vi "CRYO_MASTER_FULL_RUN3.vi"() -> ()   [LabVIEW 2017]
uses:
  LSI218Data.lvclass
  LSI336Data.lvclass
  USBData.lvclass
  6240AData.lvclass
  DMMsData.lvclass
  LMData.lvclass
  <vilib>/DAQmx/miscellaneous.llb/DAQmx Fill In Error Info.vi
  <vilib>/DAQmx/create/channels.llb/DAQmx Create Channel (DO-Digital Output).vi
  <vilib>/DAQmx/create/channels.llb/DAQmx Create Channel (AO-Voltage-Basic).vi
  <vilib>/express/express arith-compare/Formula/XNode/ExpressFormulaBlockNode.xnode
  <vilib>/Analysis/NI_AALBase.lvlib
  istr.lib/Agilent 33XXX Series/Agilent 33XXX Series.lvlib
panel:
  in  "Automatic \nScreenshots?":bool=TRUE
  in  "Frontpanel screenshots":bool
  in  "Screenshots interval":i64=3605
  in  "Record interval":i64=20
  out "Cycle #":u32=1
  in  "Measurement Interval (s)":dbl=1.0
  in  "Stop Button":bool
  in  "?":T1(tab)=enum."MEASUREMENT"
  out "RUN Identifier":string="20210209_084357_RUNIII"
  in  "Base Path (screenshots)":path=path "C:/LabVIEW/DATA/Google/TUCAN Experiments/KEK_cryotests_2019-2020/data/screenshots"
  out "error out (USB6210/6218 AOUT)":errorcluster
  in  "AOUT Labels":string[](array[string])=["PWR400H_I", "PMC183A_I"]
  in  "DOUT Labels":string[](array[string])=["D_V1_NO", "D_V2_NC", "D_CV1", "D_H1"]
  in  "AOUT assignment":tag[](array[tag])=["Dev1/ao0", "Dev1/ao1"]
  out "AO task out":refnum<k21>="20210209_084357_RUNIII_AO"
  in  "Analog Out ON?":bool=TRUE
  in  "InstName (USB6218)":string="USB6218"
  in  "USB6218 Config":T2(array[cluster])=[{"Label"="F_1", "FileFormat"="%5.5f", "Active?"=TRUE, "Physical CH"="Dev1/ai0", " terminal\n type"=10083, "ConversionType"={"Type"=enum."SimpleProp", "ConversionParameters"=[0.0, 5.0, 0.0, 500.0]}, "VoltageLimits"=[0.0, 5.0]}, {"Label"="F_2", "FileFormat"="%5.5f", "Active?"=TRUE, "Physical CH"="Dev1/ai1", " terminal\n type"=10083, "ConversionType"={"Type"=enum."SimpleProp", "ConversionParameters"=[0.0, 5.0, 0.0, 200.0]}, "VoltageLimits"=[0.0, 5.0]}, {"Label"="F_3", "FileFormat"="%5.5f", "Active?"=TRUE, "Physical CH"="Dev1/ai2", " terminal\n type"=10083, "ConversionType"={"Type"=enum."SimpleProp", "ConversionParameters"=[0.0, 5.0, 0.0, 200.0]}, "VoltageLimits"=[0.0, 5.0]}, {"Label"="F_4", "FileFormat"="%5.5f", "Active?"=TRUE, "Physical CH"="Dev1/ai3", " terminal\n type"=10083, "ConversionType"={"Type"=enum."SimpleProp", "ConversionParameters"=[0.0, 5.0, 0.0, 500.0]}, "VoltageLimits"=[0.0, 5.0]}, {"Label"="F_5", "FileFormat"="%5.5f", "Active?"=TRUE, "Physical CH"="Dev1/ai4", " terminal\n type"=10083, "ConversionType"={"Type"=enum."SimpleProp", "ConversionParameters"=[0.0, 5.0, 0.0, 500.0]}, "VoltageLimits"=[0.0, 5.0]}, {"Label"="I_CV", "FileFormat"="%3.5f", "Active?"=TRUE, "Physical CH"="Dev1/ai5", " terminal\n type"=10083, "ConversionType"={"Type"=enum."Raw", "ConversionParameters"=[0.0, 0.0, 0.0, 0.0]}, "VoltageLimits"=[0.0, 10.0]}, {"Label"="CV1_answer", "FileFormat"="%3.5f", "Active?"=TRUE, "Physical CH"="Dev1/ai6", " terminal\n type"=10083, "ConversionType"={"Type"=enum."SimpleProp", "ConversionParameters"=[1.0, 5.0, 0.0, 100.0]}, "VoltageLimits"=[0.0, 5.0]}, {"Label"="P_Dewar", "FileFormat"="%5.5e", "Active?"=TRUE, "Physical CH"="Dev1/ai7", " terminal\n type"=10083, "ConversionType"={"Type"=enum."SimpleProp", "ConversionParameters"=[1.0, 5.0, 0.0, 200000.0]}, "VoltageLimits"=[0.0, 5.0]}, {"Label"="L_Dewar", "FileFormat"="%5.5f", "Active?"=TRUE, "Physical CH"="Dev1/ai8", " terminal\n type"=10083, "ConversionType"={"Type"=enum."SimpleProp", "ConversionParameters"=[0.0, 10.0, 0.0, 100.0]}, "VoltageLimits"=[0.0, 10.0]}] {"terminal\n type" items=["Default"=-1, "RSE"=10083, "NRSE"=10078, "Differential"=10106, "Pseudodifferential"=12529]}
  out "error out (USB6218)":errorcluster
  out "error out (USB6210/6218 DOUT)":errorcluster
  out "DOUT task out":refnum<k21>="20210209_084357_DO"
  in  "DOUT Physical CH":tag[](array[tag])=["Dev1/port1/line0", "Dev1/port1/line1", "Dev1/port1/line2", "Dev1/port1/line3"]
  in  "Digital Out ON?":bool=TRUE
  in  "USB6210 Config":T2(array[cluster])=[{"Label"="P_ins", "FileFormat"="%5.5e", "Active?"=TRUE, "Physical CH"="Dev2/ai0", " terminal\n type"=10083, "ConversionType"={"Type"=enum."CC-10_LOG", "ConversionParameters"=[0.5, 9.0, 0.0, 1.0]}, "VoltageLimits"=[0.0, 10.0]}, {"Label"="P_4Kres", "FileFormat"="%5.5e", "Active?"=TRUE, "Physical CH"="Dev2/ai1", " terminal\n type"=10083, "ConversionType"={"Type"=enum."SimpleProp", "ConversionParameters"=[1.0, 5.0, 0.0, 200000.0]}, "VoltageLimits"=[0.0, 5.0]}, {"Label"="P_3HeIN", "FileFormat"="%5.5e", "Active?"=TRUE, "Physical CH"="Dev2/ai2", " terminal\n type"=10083, "ConversionType"={"Type"=enum."SimpleProp", "ConversionParameters"=[1.0, 5.0, 0.0, 200000.0]}, "VoltageLimits"=[0.0, 5.0]}, {"Label"="P_SldRTN", "FileFormat"="%5.5e", "Active?"=TRUE, "Physical CH"="Dev2/ai3", " terminal\n type"=10083, "ConversionType"={"Type"=enum."SimpleProp", "ConversionParameters"=[1.0, 5.0, 0.0, 200000.0]}, "VoltageLimits"=[0.0, 5.0]}, {"Label"="P_3Hepot", "FileFormat"="%5.5e", "Active?"=TRUE, "Physical CH"="Dev2/ai4", " terminal\n type"=10083, "ConversionType"={"Type"=enum."SimpleProp", "ConversionParameters"=[0.0, 10.0, 0.0, 133320.0]}, "VoltageLimits"=[0.0, 10.0]}, {"Label"="P_1Kpot", "FileFormat"="%5.5e", "Active?"=TRUE, "Physical CH"="Dev2/ai5", " terminal\n type"=10083, "ConversionType"={"Type"=enum."SimpleProp", "ConversionParameters"=[0.0, 10.0, 0.0, 133320.0]}, "VoltageLimits"=[0.0, 10.0]}, {"Label"="P_Dewar(old)", "FileFormat"="%5.5e", "Active?"=FALSE, "Physical CH"="Dev2/ai6", " terminal\n type"=10083, "ConversionType"={"Type"=enum."SimpleProp", "ConversionParameters"=[1.0, 5.0, 0.0, 200000.0]}, "VoltageLimits"=[0.0, 5.0]}, {"Label"="DP_HEX4", "FileFormat"="%5.5e", "Active?"=TRUE, "Physical CH"="Dev2/ai7", " terminal\n type"=10083, "ConversionType"={"Type"=enum."SimpleProp", "ConversionParameters"=[1.0, 5.0, 0.0, 1000.0]}, "VoltageLimits"=[0.0, 5.0]}, {"Label"="DP_HEX5", "FileFormat"="%5.5e", "Active?"=TRUE, "Physical CH"="Dev2/ai8", " terminal\n type"=10083, "ConversionType"={"Type"=enum."SimpleProp", "ConversionParameters"=[1.0, 5.0, 0.0, 1000.0]}, "VoltageLimits"=[0.0, 5.0]}, {"Label"="L1(old)", "FileFormat"="%5.5f", "Active?"=TRUE, "Physical CH"="Dev2/ai9", " terminal\n type"=10083, "ConversionType"={"Type"=enum."SimpleProp", "ConversionParameters"=[0.0, 10.0, 0.0, 100.0]}, "VoltageLimits"=[0.0, 10.0]}, {"Label"="L2-1", "FileFormat"="%5.5f", "Active?"=TRUE, "Physical CH"="Dev2/ai10", " terminal\n type"=10083, "ConversionType"={"Type"=enum."SimpleProp", "ConversionParameters"=[0.0, 10.0, 0.0, 100.0]}, "VoltageLimits"=[0.0, 10.0]}, {"Label"="L2-2", "FileFormat"="%5.5f", "Active?"=TRUE, "Physical CH"="Dev2/ai11", " terminal\n type"=10083, "ConversionType"={"Type"=enum."SimpleProp", "ConversionParameters"=[0.0, 10.0, 0.0, 100.0]}, "VoltageLimits"=[0.0, 10.0]}, {"Label"="L3", "FileFormat"="%5.5f", "Active?"=TRUE, "Physical CH"="Dev2/ai12", " terminal\n type"=10083, "ConversionType"={"Type"=enum."SimpleProp", "ConversionParameters"=[0.0, 10.0, 0.0, 100.0]}, "VoltageLimits"=[0.0, 10.0]}, {"Label"="P_HEX7OUT", "FileFormat"="%5.5e", "Active?"=TRUE, "Physical CH"="Dev2/ai13", " terminal\n type"=10083, "ConversionType"={"Type"=enum."SimpleProp", "ConversionParameters"=[1.0, 5.0, 0.0, 200000.0]}, "VoltageLimits"=[0.0, 5.0]}, {"Label"="P_IP", "FileFormat"="%5.5e", "Active?"=TRUE, "Physical CH"="Dev2/ai14", " terminal\n type"=10083, "ConversionType"={"Type"=enum."CC-10_LOG", "ConversionParameters"=[0.5, 9.0, 0.0, 1.0]}, "VoltageLimits"=[0.0, 10.0]}, {"Label"="V_H1", "FileFormat"="%3.5f", "Active?"=TRUE, "Physical CH"="Dev2/ai15", " terminal\n type"=10083, "ConversionType"={"Type"=enum."Raw", "ConversionParameters"=[0.0, 1.0, 0.0, 1.0]}, "VoltageLimits"=[0.0, 10.0]}] {"terminal\n type" items=["Default"=-1, "RSE"=10083, "NRSE"=10078, "Differential"=10106, "Pseudodifferential"=12529]}
  in  "RUN label":string="RUNIII"
  in  "Base Path":path=path "C:/LabVIEW/DATA/RUN_3"
  in  "InstName (USB6210)":string="USB6210"
  out "error out (USB6210)":errorcluster
  out "File Refn USB AO":refnum<file>
  out "File Refn USB DO":refnum<file>
  in  "LM measurement interval (>0)":i64=1
  in  "Active? (HP34401 LM)":bool=TRUE
  in  "Labels (HP34401 LM)":string[](array[string])=["R_L1", "L1"]
  in  "FileFormat (HP34401 LM)":string[](array[string])=["%.4f", "%.4f"]
  in  "VISA (HP34401 LM)":refnum<visa-resource-name>="GPIB0::24::INSTR"
  in  "LevelCalibration (R0, R1, L0, L1)":dbl[](array[numeric])=[179.74, 0.0, 0.0, 100.0]
  in  "InstName (HP34401 LM)":string="HP34401LM"
  out "error out (LSI336)":errorcluster
  in  "InstName (LSI336)":string="LSI336"
  in  "FileFormat (336)":string="%4.4f"
  in  "LSI336Settings(X,Y)":T3(array[cluster])=[{"LSIName"="LSi336X", "Labels"=["T1K3-1", "T1K3-2", "T3He5", "T3He8"], "SensorLocations"=[enum."T1K3-1", enum."T1K3-2", enum."T3He5", enum."T3He8"], "Active?"=TRUE, "VISA res. name"="COM15_LSI336Y"}, {"LSIName"="LSi336Y", "Labels"=["T3He6-1", "T3He6-2", "T3He7-1", "T3He7-2"], "SensorLocations"=[enum."T3He6-1", enum."T3He6-2", enum."T3He7-1", enum."T3He7-2"], "Active?"=TRUE, "VISA res. name"="COM20_LSI336X"}]
  in  "FileFormat (218)":string="%4.4f"
  in  "InstName (LSI218)":string="LSI218"
  in  "LSI218Settings(A-F)":T3(array[cluster])=[{"LSIName"="LSI218A", "Labels"=["T3He10", "T3He1-1", "TTH3", "TTH4", "TTH1", "TTH2", "T4He1", "T1K1"], "SensorLocations"=[enum."T3He10", enum."T3He1-1", enum."TTH3", enum."TTH4", enum."TTH1", enum."TTH2", enum."T4He1", enum."T1K1"], "Active?"=TRUE, "VISA res. name"="GPIB0::7::INSTR"}, {"LSIName"="LSI218B", "Labels"=["N.C.", "N.C.", "N.C.", "N.C.", "T3He2-1", "T3He2-2", "T3He3", "T3He1-4"], "SensorLocations"=[enum."N.C.", enum."N.C.", enum."N.C.", enum."N.C.", enum."T3He2-1", enum."T3He2-2", enum."T3He3", enum."T3He1-4"], "Active?"=TRUE, "VISA res. name"="GPIB0::4::INSTR"}, {"LSIName"="LSI218C", "Labels"=["T4He3-1", "T4He3-2", "T4He3-3", "T4He3-4", "T4He2-1", "T4He2-2", "T4He4", "T4He5"], "SensorLocations"=[enum."T4He3-1", enum."T4He3-2", enum."T4He3-3", enum."T4He3-4", enum."T4He2-1", enum."T4He2-2", enum."T4He4", enum."T4He5"], "Active?"=TRUE, "VISA res. name"="GPIB0::3::INSTR"}, {"LSIName"="LSI218D", "Labels"=["T4He6", "T4He9", "T3He1-2", "T3He1-3", "T4He7", "T4He8", "T4He10", "T1K6"], "SensorLocations"=[enum."T4He6", enum."T4He9", enum."T3He1-2", enum."T3He1-3", enum."T4He7", enum."T4He8", enum."T4He10", enum."T1K6"], "Active?"=TRUE, "VISA res. name"="GPIB0::5::INSTR"}, {"LSIName"="LSI218E", "Labels"=["TIP1", "N.C.", "TIP2", "N.C.", "TIP3", "TIP4", "TIP5", "N.C."], "SensorLocations"=[enum."TIP1", enum."N.C.", enum."TIP2", enum."N.C.", enum."TIP3", enum."TIP4", enum."TIP5", enum."N.C."], "Active?"=TRUE, "VISA res. name"="GPIB0::11::INSTR"}, {"LSIName"="LSI218F", "Labels"=["T1K2", "T1K4", "T1K5", "T3He4", "T3He9", "TIP6", "N.C.", "N.C."], "SensorLocations"=[enum."T1K2", enum."T1K4", enum."T1K5", enum."T3He4", enum."T3He9", enum."TIP6", enum."N.C.", enum."N.C."], "Active?"=TRUE, "VISA res. name"="GPIB0::8::INSTR"}]
  out "error out (LSI218)":errorcluster={"status"=TRUE, "code"=-1073807338, "source"="VISA Close in Lake Shore Cryotronics 218.lvlib:Close.vi->LSI218Data.lvclass:LSI218Data_terminate.vi->CRYO_MASTER_FULL_RUN3.vi"}
  out "RUN Identifier 2":string="20210209_084357_RUNIII" caption="RUN Identifier"
  out "error out (HP34401 LM)":errorcluster
  out "Graph 3":T4(graph)=[{"TimeArray"=[timestamp(3695672639.4136896 s since 1904-01-01)], "DataArray"=[-0.36185606613019977]}, {"TimeArray"=[timestamp(3695672639.4136896 s since 1904-01-01)], "DataArray"=[-1.4204433335631088]}, {"TimeArray"=[timestamp(3695672639.4136896 s since 1904-01-01)], "DataArray"=[0.28794373208354185]}, {"TimeArray"=[timestamp(3695672639.4136896 s since 1904-01-01)], "DataArray"=[-3.0973798990583647]}, {"TimeArray"=[timestamp(3695672639.4136896 s since 1904-01-01)], "DataArray"=[18.382396544680894]}, {"TimeArray"=[timestamp(3695672639.4136896 s since 1904-01-01)], "DataArray"=[-0.0024966396874153696]}, {"TimeArray"=[timestamp(3695672639.4136896 s since 1904-01-01)], "DataArray"=[107.20664477077275]}] caption="XY Graph"
  out "Graph 1":T4(graph)=[{"TimeArray"=[timestamp(3695672639.4087214 s since 1904-01-01)], "DataArray"=[18.674861858538797]}, {"TimeArray"=[timestamp(3695672639.4087214 s since 1904-01-01)], "DataArray"=[97865.81349287118]}, {"TimeArray"=[timestamp(3695672639.4087214 s since 1904-01-01)], "DataArray"=[100998.44453584745]}, {"TimeArray"=[timestamp(3695672639.4087214 s since 1904-01-01)], "DataArray"=[100709.02551899779]}, {"TimeArray"=[timestamp(3695672639.4087214 s since 1904-01-01)], "DataArray"=[101407.09548804205]}, {"TimeArray"=[timestamp(3695672639.4087214 s since 1904-01-01)], "DataArray"=[101279.08758660906]}, {"TimeArray"=[timestamp(3695672639.4087214 s since 1904-01-01)], "DataArray"=[0.0]}, {"TimeArray"=[timestamp(3695672639.4087214 s since 1904-01-01)], "DataArray"=[100273.25274306418]}, {"TimeArray"=[timestamp(3695672639.4087214 s since 1904-01-01)], "DataArray"=[4.684755546764993e-05]}, {"TimeArray"=[timestamp(3695672639.4136896 s since 1904-01-01)], "DataArray"=[102243.79868545999]}] caption="XY Graph"
  in  "FIle suffix 4":string="Graph4_noise"
  in  "Take Screenshot! 4":bool
  in  "Take Screenshot! 3":bool
  in  "Take Screenshot! 2":bool
  in  "Take Screenshot! 1":bool
  in  "FIle suffix 3":string="Graph3_noise"
  in  "FIle suffix 2":string="Graph2_noise"
  in  "FIle suffix 1":string="Graph1_noise"
  in  "log/linear 2":bool
  in  "Tab Control 2":T5(tab)
  in  "Plot selecter (USB6210)\n    1      2     3     4":bool[][](array[boolean])=[[TRUE, FALSE, FALSE, FALSE], [TRUE, FALSE, FALSE, FALSE], [TRUE, FALSE, FALSE, FALSE], [TRUE, FALSE, FALSE, FALSE], [TRUE, FALSE, FALSE, FALSE], [TRUE, FALSE, FALSE, FALSE], [TRUE, FALSE, FALSE, FALSE], [FALSE, TRUE, FALSE, FALSE], [FALSE, TRUE, FALSE, FALSE], [FALSE, TRUE, FALSE, FALSE], [FALSE, TRUE, FALSE, FALSE], [FALSE, TRUE, FALSE, FALSE], [FALSE, TRUE, FALSE, FALSE], [TRUE, FALSE, FALSE, FALSE], [TRUE, FALSE, FALSE, FALSE], [FALSE, FALSE, FALSE, FALSE]]
  out "All Labels (USB6210)":string[](array[string])=["P_ins", "P_4Kres", "P_3HeIN", "P_SldRTN", "P_3Hepot", "P_1Kpot", "P_Dewar(old)", "DP_HEX4", "DP_HEX5", "L1(old)", "L2-1", "L2-2", "L3", "P_HEX7OUT", "P_IP", "V_H1"]
  out "Last Data \n(USB6210)":dbl[](array[numeric])=[18.674861858538797, 97865.81349287118, 100998.44453584745, 100709.02551899779, 101407.09548804205, 101279.08758660906, 0.0, -48.20456535494683, 0.06691412080322978, 10.108489682314854, 0.1698011167381339, -0.07483544992953703, 0.04024895650740204, 100273.25274306418, 4.684755546764993e-05, 5.953981760223165] format="%#_6e"
  out "Time of Last Measurement (USB6210)":timestamp=timestamp(3695672639.4087214 s since 1904-01-01)
  out "USB6210 Status":T6(ring)=enum."Ready"
  out "Last Vol\n(USB6210)":dbl[](array[numeric])=[8.135628698970727, 2.9573162698574236, 3.019968890716949, 3.0141805103799557, 7.606292790882241, 7.596691238119492, 0.0, 0.8071817385802127, 1.000267656483213, 1.0108489682314854, 0.01698011167381339, -0.007483544992953703, 0.004024895650740204, 3.0054650548612836, 5.335343467039768, 5.953981760223165] format="%_5f"
  out "Labels (HP34401 LM) 2":string[](array[string])=["R_L1", "L1"]
  out "LastData (HP34401 LM)":dbl[](array[numeric])=[166.68232, 7.2647602091910555]
  in  "Plot selecter (HP34401A)\n    1      2     3     4":bool[][](array[boolean])=[[FALSE, TRUE, FALSE, FALSE], [FALSE, TRUE, FALSE, FALSE], [TRUE, FALSE, FALSE, FALSE], [TRUE, FALSE, FALSE, FALSE], [TRUE, FALSE, FALSE, FALSE], [TRUE, FALSE, FALSE, FALSE], [TRUE, FALSE, FALSE, FALSE], [FALSE, TRUE, FALSE, FALSE], [FALSE, TRUE, FALSE, FALSE], [FALSE, TRUE, FALSE, FALSE], [FALSE, TRUE, FALSE, FALSE], [FALSE, TRUE, FALSE, FALSE], [FALSE, TRUE, FALSE, FALSE], [TRUE, FALSE, FALSE, FALSE], [TRUE, FALSE, FALSE, FALSE], [FALSE, FALSE, FALSE, FALSE]]
  out "Time of Last Measurement (USB6218)":timestamp=timestamp(3695672639.4136896 s since 1904-01-01)
  out "USB6218 Status":T6(ring)=enum."Ready"
  out "Last Vol \n(USB6218)":dbl[](array[numeric])=[-0.003618560661301998, -0.03551108333907772, 0.0071985933020885465, -0.030973798990583647, 0.18382396544680896, -0.0024966396874153696, -0.0029609827608362395, 3.0448759737091997, 10.720664477077275] format="%_5f"
  out "Last Data \n(USB6218)":dbl[](array[numeric])=[-0.36185606613019977, -1.4204433335631088, 0.28794373208354185, -3.0973798990583647, 18.382396544680894, -0.0024966396874153696, -25.07402456902091, 102243.79868545999, 107.20664477077275] format="%#_6e"
  out "All Labels (USB6218)":string[](array[string])=["F_1", "F_2", "F_3", "F_4", "F_5", "I_CV", "CV1_answer", "P_Dewar", "L_Dewar"]
  in  "Plot selecter (USB6218)\n    1      2     3     4":bool[][](array[boolean])=[[FALSE, FALSE, TRUE, FALSE], [FALSE, FALSE, TRUE, FALSE], [FALSE, FALSE, TRUE, FALSE], [FALSE, FALSE, TRUE, FALSE], [FALSE, FALSE, TRUE, FALSE], [FALSE, FALSE, TRUE, FALSE], [FALSE, FALSE, FALSE, FALSE], [TRUE, FALSE, FALSE, FALSE], [FALSE, FALSE, TRUE, FALSE], [FALSE, FALSE, FALSE, TRUE], [FALSE, FALSE, FALSE, TRUE], [FALSE, FALSE, FALSE, TRUE], [FALSE, FALSE, FALSE, TRUE], [FALSE, FALSE, FALSE, FALSE], [FALSE, FALSE, FALSE, FALSE], [FALSE, FALSE, FALSE, FALSE]]
  out "Time of Last Measurement (LSI218)":timestamp=timestamp(3695672639.4087214 s since 1904-01-01)
  out "LSI218 Status":T7(ring)=enum."Measuring"
  out "Last Data \nLSI218 (1)":dbl[](array[numeric])=[286.39, 292.79, 245.71, 242.82, 192.73, 208.05, 129.14, 157.86, 30.0, 0.0, 0.0, 0.0, 214.32, 209.26, 161.19, 290.41, 293.53, 293.65, 291.53, 291.58, 216.58, 205.59, 215.41, 218.49]
  out "Labels LSI218 (1)":string[](array[string])=["T3He10", "T3He1-1", "TTH3", "TTH4", "TTH1", "TTH2", "T4He1", "T1K1", "N.C.", "N.C.", "N.C.", "N.C.", "T3He2-1", "T3He2-2", "T3He3", "T3He1-4", "T4He3-1", "T4He3-2", "T4He3-3", "T4He3-4", "T4He2-1", "T4He2-2", "T4He4", "T4He5"]
  in  "Plot selecter LSI218(1)\n    1      2     3     4":bool[][](array[boolean])=[[FALSE, FALSE, FALSE, FALSE], [FALSE, FALSE, FALSE, FALSE], [FALSE, FALSE, FALSE, TRUE], [FALSE, FALSE, FALSE, TRUE], [FALSE, FALSE, FALSE, TRUE], [FALSE, FALSE, FALSE, TRUE], [FALSE, FALSE, FALSE, TRUE], [FALSE, FALSE, FALSE, TRUE], [FALSE, FALSE, FALSE, FALSE], [FALSE, FALSE, FALSE, FALSE], [FALSE, FALSE, FALSE, FALSE], [FALSE, FALSE, FALSE, FALSE], [FALSE, FALSE, FALSE, TRUE], [FALSE, FALSE, FALSE, TRUE], [FALSE, FALSE, FALSE, FALSE], [FALSE, FALSE, FALSE, FALSE], [FALSE, FALSE, FALSE, TRUE], [FALSE, FALSE, FALSE, TRUE], [FALSE, FALSE, FALSE, TRUE], [FALSE, FALSE, FALSE, TRUE], [FALSE, FALSE, FALSE, TRUE], [FALSE, FALSE, FALSE, TRUE], [FALSE, FALSE, FALSE, TRUE], [FALSE, FALSE, FALSE, FALSE]]
  out "Active?\n (1)":bool[](array[boolean])=[TRUE, TRUE, TRUE, TRUE, TRUE, TRUE, TRUE, TRUE, TRUE, TRUE, TRUE, TRUE, TRUE, TRUE, TRUE, TRUE, TRUE, TRUE, TRUE, TRUE, TRUE, TRUE, TRUE, TRUE]
  out "Labels LSI218 (2)":string[](array[string])=["T4He6", "T4He9", "T3He1-2", "T3He1-3", "T4He7", "T4He8", "T4He10", "T1K6", "TIP1", "N.C.", "TIP2", "N.C.", "TIP3", "TIP4", "TIP5", "N.C.", "T1K2", "T1K4", "T1K5", "T3He4", "T3He9", "TIP6", "N.C.", "N.C."]
  out "Active?\n(2)":bool[](array[boolean])=[TRUE, TRUE, TRUE, TRUE, TRUE, TRUE, TRUE, TRUE, TRUE, TRUE, TRUE, TRUE, TRUE, TRUE, TRUE, TRUE, TRUE, TRUE, TRUE, TRUE, TRUE, TRUE, TRUE, TRUE]
  out "Last Data \nLSI218 (2)":dbl[](array[numeric])=[214.17, 227.11, 292.96, 290.69, 256.79, 281.72, 274.72, 287.38, 279.49, 0.0, 232.53, 688.49, 216.83, 149.55, 173.98, 688.58, 178.46, 128.79, 144.74, 152.95, 140.88, 150.1, 0.433, 0.0]
  in  "Plot selecter LSI218(2)\n    1      2     3     4":bool[][](array[boolean])=[[FALSE, FALSE, FALSE, FALSE], [FALSE, FALSE, FALSE, FALSE], [FALSE, FALSE, FALSE, FALSE], [FALSE, FALSE, FALSE, FALSE], [FALSE, FALSE, FALSE, FALSE], [FALSE, FALSE, FALSE, FALSE], [FALSE, FALSE, FALSE, FALSE], [FALSE, FALSE, FALSE, FALSE], [FALSE, FALSE, FALSE, FALSE], [FALSE, FALSE, FALSE, FALSE], [FALSE, FALSE, FALSE, FALSE], [FALSE, FALSE, FALSE, FALSE], [FALSE, FALSE, FALSE, FALSE], [FALSE, FALSE, FALSE, FALSE], [FALSE, FALSE, FALSE, FALSE], [FALSE, FALSE, FALSE, FALSE], [FALSE, FALSE, FALSE, TRUE], [FALSE, FALSE, FALSE, TRUE], [FALSE, FALSE, FALSE, TRUE], [FALSE, FALSE, FALSE, TRUE], [FALSE, FALSE, FALSE, FALSE], [FALSE, FALSE, FALSE, FALSE], [FALSE, FALSE, FALSE, FALSE], [FALSE, FALSE, FALSE, FALSE]]
  in  "Plot selecter LSI336 \n     1      2     3     4":bool[][](array[boolean])=[[FALSE, FALSE, FALSE, TRUE], [FALSE, FALSE, FALSE, TRUE], [FALSE, FALSE, FALSE, TRUE], [FALSE, FALSE, FALSE, TRUE], [FALSE, FALSE, FALSE, TRUE], [FALSE, FALSE, FALSE, TRUE], [FALSE, FALSE, FALSE, TRUE], [FALSE, FALSE, FALSE, TRUE]]
  out "Time of Last Measurement (LSI336)":timestamp=timestamp(3695672639.4087214 s since 1904-01-01)
  out "Last Data \nLSI336":dbl[](array[numeric])=[117.963, 117.927, 169.419, 129.275, 167.919, 163.1, 162.659, 160.848]
  out "Active?\n(LSI336)":bool[](array[boolean])=[TRUE, TRUE, TRUE, TRUE, TRUE, TRUE, TRUE, TRUE]
  out "Labels LSI336":string[](array[string])=["T1K3-1", "T1K3-2", "T3He5", "T3He8", "T3He6-1", "T3He6-2", "T3He7-1", "T3He7-2"]
  out "LSI336 Status":T7(ring)=enum."Measuring"
  in  "log/linear 1":bool
  out "Graph 2":T4(graph)=[{"TimeArray"=[timestamp(3695672639.4087214 s since 1904-01-01)], "DataArray"=[-48.20456535494683]}, {"TimeArray"=[timestamp(3695672639.4087214 s since 1904-01-01)], "DataArray"=[0.06691412080322978]}, {"TimeArray"=[timestamp(3695672639.4087214 s since 1904-01-01)], "DataArray"=[10.108489682314854]}, {"TimeArray"=[timestamp(3695672639.4087214 s since 1904-01-01)], "DataArray"=[0.1698011167381339]}, {"TimeArray"=[timestamp(3695672639.4087214 s since 1904-01-01)], "DataArray"=[-0.07483544992953703]}, {"TimeArray"=[timestamp(3695672639.4087214 s since 1904-01-01)], "DataArray"=[0.04024895650740204]}, {"TimeArray"=[timestamp(3695672639.4087214 s since 1904-01-01)], "DataArray"=[166.68232]}, {"TimeArray"=[timestamp(3695672639.4087214 s since 1904-01-01)], "DataArray"=[7.2647602091910555]}] caption="XY Graph"
  out "Graph 4":T4(graph)=[{"TimeArray"=[timestamp(3695672639.4087214 s since 1904-01-01)], "DataArray"=[245.71]}, {"TimeArray"=[timestamp(3695672639.4087214 s since 1904-01-01)], "DataArray"=[242.82]}, {"TimeArray"=[timestamp(3695672639.4087214 s since 1904-01-01)], "DataArray"=[192.73]}, {"TimeArray"=[timestamp(3695672639.4087214 s since 1904-01-01)], "DataArray"=[208.05]}, {"TimeArray"=[timestamp(3695672639.4087214 s since 1904-01-01)], "DataArray"=[129.14]}, {"TimeArray"=[timestamp(3695672639.4087214 s since 1904-01-01)], "DataArray"=[157.86]}, {"TimeArray"=[timestamp(3695672639.4087214 s since 1904-01-01)], "DataArray"=[214.32]}, {"TimeArray"=[timestamp(3695672639.4087214 s since 1904-01-01)], "DataArray"=[209.26]}, {"TimeArray"=[timestamp(3695672639.4087214 s since 1904-01-01)], "DataArray"=[293.53]}, {"TimeArray"=[timestamp(3695672639.4087214 s since 1904-01-01)], "DataArray"=[293.65]}, {"TimeArray"=[timestamp(3695672639.4087214 s since 1904-01-01)], "DataArray"=[291.53]}, {"TimeArray"=[timestamp(3695672639.4087214 s since 1904-01-01)], "DataArray"=[291.58]}, {"TimeArray"=[timestamp(3695672639.4087214 s since 1904-01-01)], "DataArray"=[216.58]}, {"TimeArray"=[timestamp(3695672639.4087214 s since 1904-01-01)], "DataArray"=[205.59]}, {"TimeArray"=[timestamp(3695672639.4087214 s since 1904-01-01)], "DataArray"=[215.41]}, {"TimeArray"=[timestamp(3695672639.4087214 s since 1904-01-01)], "DataArray"=[178.46]}, {"TimeArray"=[timestamp(3695672639.4087214 s since 1904-01-01)], "DataArray"=[128.79]}, {"TimeArray"=[timestamp(3695672639.4087214 s since 1904-01-01)], "DataArray"=[144.74]}, {"TimeArray"=[timestamp(3695672639.4087214 s since 1904-01-01)], "DataArray"=[152.95]}, {"TimeArray"=[timestamp(3695672639.4087214 s since 1904-01-01)], "DataArray"=[117.963]}, {"TimeArray"=[timestamp(3695672639.4087214 s since 1904-01-01)], "DataArray"=[117.927]}, {"TimeArray"=[timestamp(3695672639.4087214 s since 1904-01-01)], "DataArray"=[169.419]}, {"TimeArray"=[timestamp(3695672639.4087214 s since 1904-01-01)], "DataArray"=[129.275]}, {"TimeArray"=[timestamp(3695672639.4087214 s since 1904-01-01)], "DataArray"=[167.919]}, {"TimeArray"=[timestamp(3695672639.4087214 s since 1904-01-01)], "DataArray"=[163.1]}, {"TimeArray"=[timestamp(3695672639.4087214 s since 1904-01-01)], "DataArray"=[162.659]}, {"TimeArray"=[timestamp(3695672639.4087214 s since 1904-01-01)], "DataArray"=[160.848]}] caption="XY Graph"
  in  "log/linear 4":bool
  in  "log/linear 3":bool
  out "RUN Identifier 3":string="20210209_084357_RUNIII" caption="RUN Identifier"
  in  "AutoFill Source (P)":T8(ring)=enum."USB6218AI"
  in  "AutoFill Source (L)":T8(ring)
  out "RUN Identifier 4":string="20210209_084357_RUNIII" caption="RUN Identifier"
  out "Fill (false)":bool=TRUE
  in  "Fill state":bool
  out "state 1 (false)":bool=TRUE
  out "state 1":bool
  out "state 2":bool
  out "state 2 (false)":bool=TRUE
  out "Status V2 CTRL":enum16{"Pressurize", "Release"}(ring)=enum."Release"
  out "Status V1 CTRL":enum16{"Pressurize", "Release"}(ring)
  out "Lav (%)":dbl=43.184746563343246 format="%0.2f"
  out "Lstd":dbl=0.005294410757043201 format="%0.2f"
  out "Last N M.A. Levels":dbl[](array[numeric])=[43.182022097916416, 43.178240727788925, 43.177254283449095, 43.18267972752829, 43.18366617192395, 43.184323801491566, 43.18859839376898, 43.188105171572296, 43.18498143104121, 43.18300854229432, 43.18415939405067, 43.181528875721675, 43.189256023335034, 43.19862724492309] format="%_5e"
  out "Lstd history":dbl(graph)=0.00311953003864109
  out "Lav history":dbl(graph)=43.183302126935246
  out "Target Index (L)":i32=12
  in  "Auto Fll He L. label":string="L3"
  out "Target Index (P)":i32=7
  in  "Auto Fll Dewar P. label":string="P_Dewar"
  out "He Level":T9(graph)=[{"TimeArray"=[timestamp(3695183960.9608912 s since 1904-01-01), timestamp(3695183961.957368 s since 1904-01-01), timestamp(3695183962.9580655 s since 1904-01-01), timestamp(3695183963.961592 s since 1904-01-01), timestamp(3695183964.958559 s since 1904-01-01), timestamp(3695183965.95824 s since 1904-01-01), timestamp(3695183966.9615526 s since 1904-01-01), timestamp(3695183967.9570584 s since 1904-01-01), timestamp(3695183969.170517 s since 1904-01-01), timestamp(3695183970.170328 s since 1904-01-01), timestamp(3695183971.2289977 s since 1904-01-01), timestamp(3695183972.234284 s since 1904-01-01), timestamp(3695183973.2368255 s since 1904-01-01), timestamp(3695183974.2384686 s since 1904-01-01)], "Filtered X"=[43.18185769046936, 43.17462376512705, 43.179227172287, 43.19501028222973, 43.18580346805203, 43.1772542833975, 43.19632554139665, 43.19303739344301, 43.17330850592768, 43.16936272840992, 43.20092894842209, 43.18251532012701, 43.204217096381115, 43.20684761476211]}, {"TimeArray"=[timestamp(3695183960.9608912 s since 1904-01-01), timestamp(3695183961.957368 s since 1904-01-01), timestamp(3695183962.9580655 s since 1904-01-01), timestamp(3695183963.961592 s since 1904-01-01), timestamp(3695183964.958559 s since 1904-01-01), timestamp(3695183965.95824 s since 1904-01-01), timestamp(3695183966.9615526 s since 1904-01-01), timestamp(3695183967.9570584 s since 1904-01-01), timestamp(3695183969.170517 s since 1904-01-01), timestamp(3695183970.170328 s since 1904-01-01), timestamp(3695183971.2289977 s since 1904-01-01), timestamp(3695183972.234284 s since 1904-01-01), timestamp(3695183973.2368255 s since 1904-01-01), timestamp(3695183974.2384686 s since 1904-01-01)], "Filtered X"=[43.182022097916416, 43.178240727788925, 43.177254283449095, 43.18267972752829, 43.18366617192395, 43.184323801491566, 43.18859839376898, 43.188105171572296, 43.18498143104121, 43.18300854229432, 43.18415939405067, 43.181528875721675, 43.189256023335034, 43.19862724492309]}] caption="XY Graph"
  in  "P_safelimit_high (Pa)":dbl=300000.0 format="%_4e"
  in  "P_safelimit_low (Pa)":dbl=100.0 format="%_4e"
  in  "Auto Fill ON?":bool
  out "Pstd history":dbl(graph)=65.22033190545778
  out "Pav history":dbl(graph)=109652.45552761255
  in  "Mov. Avg Interval":i64=4
  in  "V2 (N.C.)":bool
  in  "V1 (N.O.)":bool=TRUE
  in  "N for sampling":i64=7
  in  "L_low (%)":dbl=100.0 format="%_3f"
  in  "L_high (%)":dbl=100.0 format="%_3g"
  in  "P_2_low (Pa)":dbl=105000.0 format="%_4e"
  in  "P_1_low (Pa)":dbl=120000.0 format="%_4g"
  in  "P_2_high (Pa)":dbl=110000.0 format="%_4e"
  in  "P_1_high (Pa)":dbl=123000.0 format="%_4e"
  out "Dewar Pressure":T9(graph)=[{"TimeArray"=[timestamp(3695183960.9608912 s since 1904-01-01), timestamp(3695183961.957368 s since 1904-01-01), timestamp(3695183962.9580655 s since 1904-01-01), timestamp(3695183963.961592 s since 1904-01-01), timestamp(3695183964.958559 s since 1904-01-01), timestamp(3695183965.95824 s since 1904-01-01), timestamp(3695183966.9615526 s since 1904-01-01), timestamp(3695183967.9570584 s since 1904-01-01), timestamp(3695183969.170517 s since 1904-01-01), timestamp(3695183970.170328 s since 1904-01-01), timestamp(3695183971.2289977 s since 1904-01-01), timestamp(3695183972.234284 s since 1904-01-01), timestamp(3695183973.2368255 s since 1904-01-01), timestamp(3695183974.2384686 s since 1904-01-01)], "Filtered X"=[109963.7475690302, 109450.83786052199, 109450.8378612322, 109845.38379062472, 109769.7624867718, 109506.73186680171, 109649.75476646093, 109764.8306628372, 109529.74704682652, 109345.62561207346, 109794.42160760953, 109480.4288056041, 109766.4746046815, 109687.56541811737]}, {"TimeArray"=[timestamp(3695183960.9608912 s since 1904-01-01), timestamp(3695183961.957368 s since 1904-01-01), timestamp(3695183962.9580655 s since 1904-01-01), timestamp(3695183963.961592 s since 1904-01-01), timestamp(3695183964.958559 s since 1904-01-01), timestamp(3695183965.95824 s since 1904-01-01), timestamp(3695183966.9615526 s since 1904-01-01), timestamp(3695183967.9570584 s since 1904-01-01), timestamp(3695183969.170517 s since 1904-01-01), timestamp(3695183970.170328 s since 1904-01-01), timestamp(3695183971.2289977 s since 1904-01-01), timestamp(3695183972.234284 s since 1904-01-01), timestamp(3695183973.2368255 s since 1904-01-01), timestamp(3695183974.2384686 s since 1904-01-01)], "Filtered X"=[109738.52760097096, 109708.93665645414, 109668.24910755549, 109677.70177035227, 109629.20549978768, 109643.17900135761, 109692.90822766478, 109672.76994571791, 109612.7660857316, 109572.48952204952, 109608.65623233668, 109537.55576802841, 109596.73765749215, 109682.22260900313]}] caption="XY Graph"
  out "Last N M.A. Pressures":dbl[](array[numeric])=[109738.52760097096, 109708.93665645414, 109668.24910755549, 109677.70177035227, 109629.20549978768, 109643.17900135761, 109692.90822766478, 109672.76994571791, 109612.7660857316, 109572.48952204952, 109608.65623233668, 109537.55576802841, 109596.73765749215, 109682.22260900313] format="%_5e"
  out "Pav (Pa)":dbl=109645.85040603587 format="%0.4e"
  out "Pstd":dbl=55.905802738156126 format="%0.4e"
  out "File Refn DewarCTRL":refnum<file>
  out "Error Out (Dewar CTRL":errorcluster
  in  "lower limit (mA) \n(PMC)":dbl=4.0 format="%_3f"
  in  "upper limit (mA)\n (PMC)":dbl=40.0 format="%_3f"
  in  "OUTPUT\n(PMC)":bool
  in  "Set Current (mA)\n (PMC)":dbl=4.0 min=4.0 max=40.0 format="%_3g"
  in  "update values":bool
  out "Monitor Current (mA)":dbl=-0.1982033970495195 min=0.0 max=1.9 format="%_4e"
  in  "update current":bool
  out "USB 6218 AOUT":dbl[](array[numeric])=[0.004, 0.004, 0.06969546425555169, 0.06969546425555169]
  out "Graph 7":T10(graph) caption="XY Graph"
  in  "lower limit (mA) \n(PWR)":dbl=4.0 format="%_3f"
  in  "upper limit (mA)\n (PWR)":dbl=20.0 format="%_3f"
  in  "lower limit (mA)":dbl=4.0 format="%_3f"
  in  "SetCurrent 2 (mA)":dbl=4.0 min=4.0 max=500.0 format="%_3f"
  in  "upper limit (mA)":dbl=500.0 format="%_3f"
  out "error out (KIKUSI CTRL)":errorcluster
  out "ActualVoltage (V)":dbl[](array[numeric]) format="%_6g"
  out "ActualCurrent (A)":dbl[](array[numeric])=[0.004, 0.004] format="%_3e"
  in  "SetCurrent 1 (mA)":dbl=4.0 min=4.0 max=500.0 format="%_3g"
  in  "Output\n (ADCMT)":bool[](array[boolean])=[FALSE, FALSE]
  out "error out (ADCMT6420A)":errorcluster
  in  "Voltage limits (V)":dbl[](array[numeric])=[12.0, 12.0] format="%_3f"
  in  "CtrlLabels":string[](array[string])=["CV2", "CV3"]
  in  "VISA":refnum<visa-resource-name>[](array[refnum])=["GPIB0::1::INSTR", "GPIB0::12::INSTR"]
  out "Initialized?":bool
  in  "InstName":string="ADCMT6240"
  out "Graph 6":T9(graph)=[{"TimeArray"=[timestamp(3695085214.3168983 s since 1904-01-01), timestamp(3695085244.964852 s since 1904-01-01), timestamp(3695085246.0168433 s since 1904-01-01), timestamp(3695085588.0010176 s since 1904-01-01)], "Filtered X"=[0.001, 0.005, 0.005, 0.01]}, {"TimeArray"=[timestamp(3695085214.3168983 s since 1904-01-01), timestamp(3695085244.964852 s since 1904-01-01), timestamp(3695085246.0168433 s since 1904-01-01), timestamp(3695085588.0010176 s since 1904-01-01)], "Filtered X"=[0.004, 0.004, 0.004, 0.004]}, {"TimeArray"=[timestamp(3695085214.3168983 s since 1904-01-01), timestamp(3695085244.964852 s since 1904-01-01), timestamp(3695085246.0168433 s since 1904-01-01), timestamp(3695085588.0010176 s since 1904-01-01)], "Filtered X"=[0.001, 0.005, 0.005, 0.01]}, {"TimeArray"=[timestamp(3695085214.3168983 s since 1904-01-01), timestamp(3695085244.964852 s since 1904-01-01), timestamp(3695085246.0168433 s since 1904-01-01), timestamp(3695085588.0010176 s since 1904-01-01)], "Filtered X"=[0.004, 0.004, 0.004, 0.004]}] caption="XY Graph"
  in  "Initialize":bool